vi "Velociprobe_Nanopositioner_Control_RT_2.vi"() -> ()   [LabVIEW 2015] (continued)
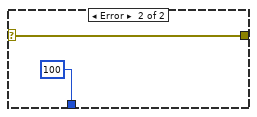
[diagram p2: hidden frame]
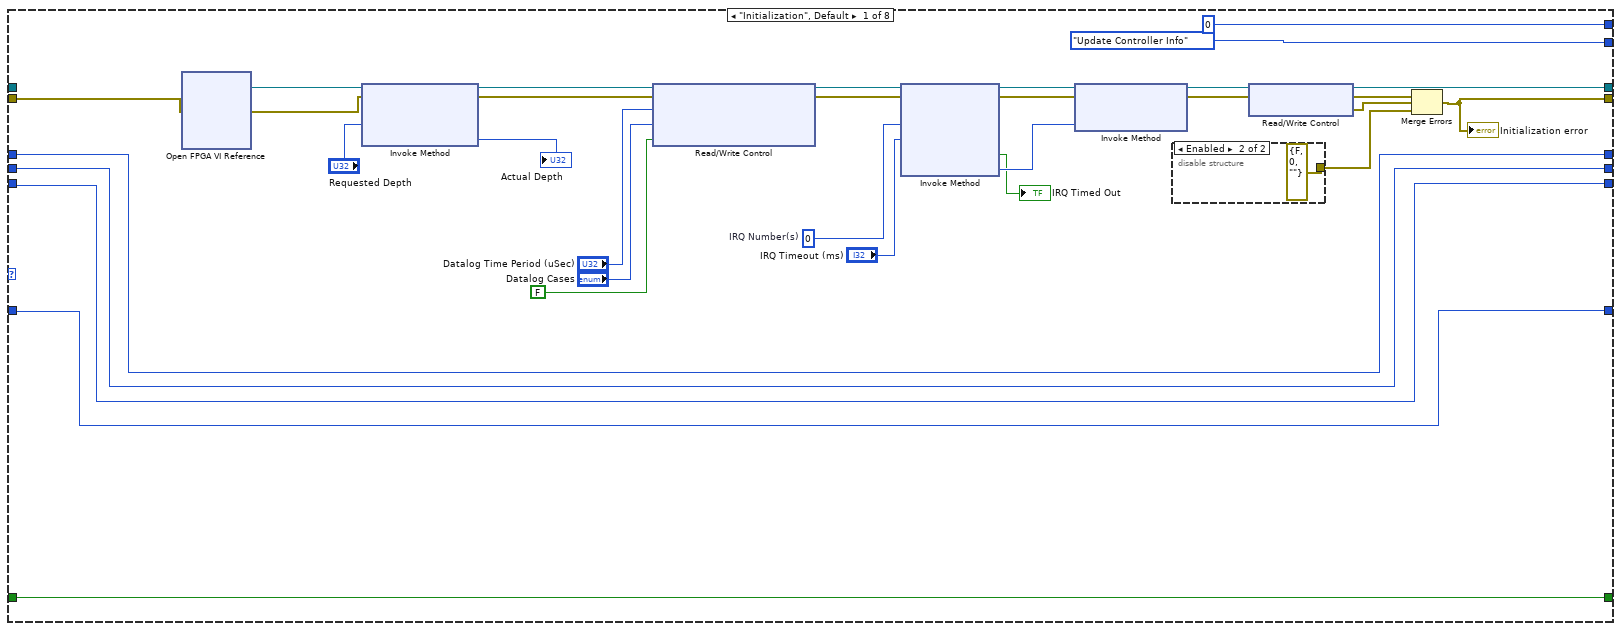
[diagram p3: hidden frame]
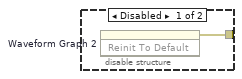
[diagram p4: hidden frame]
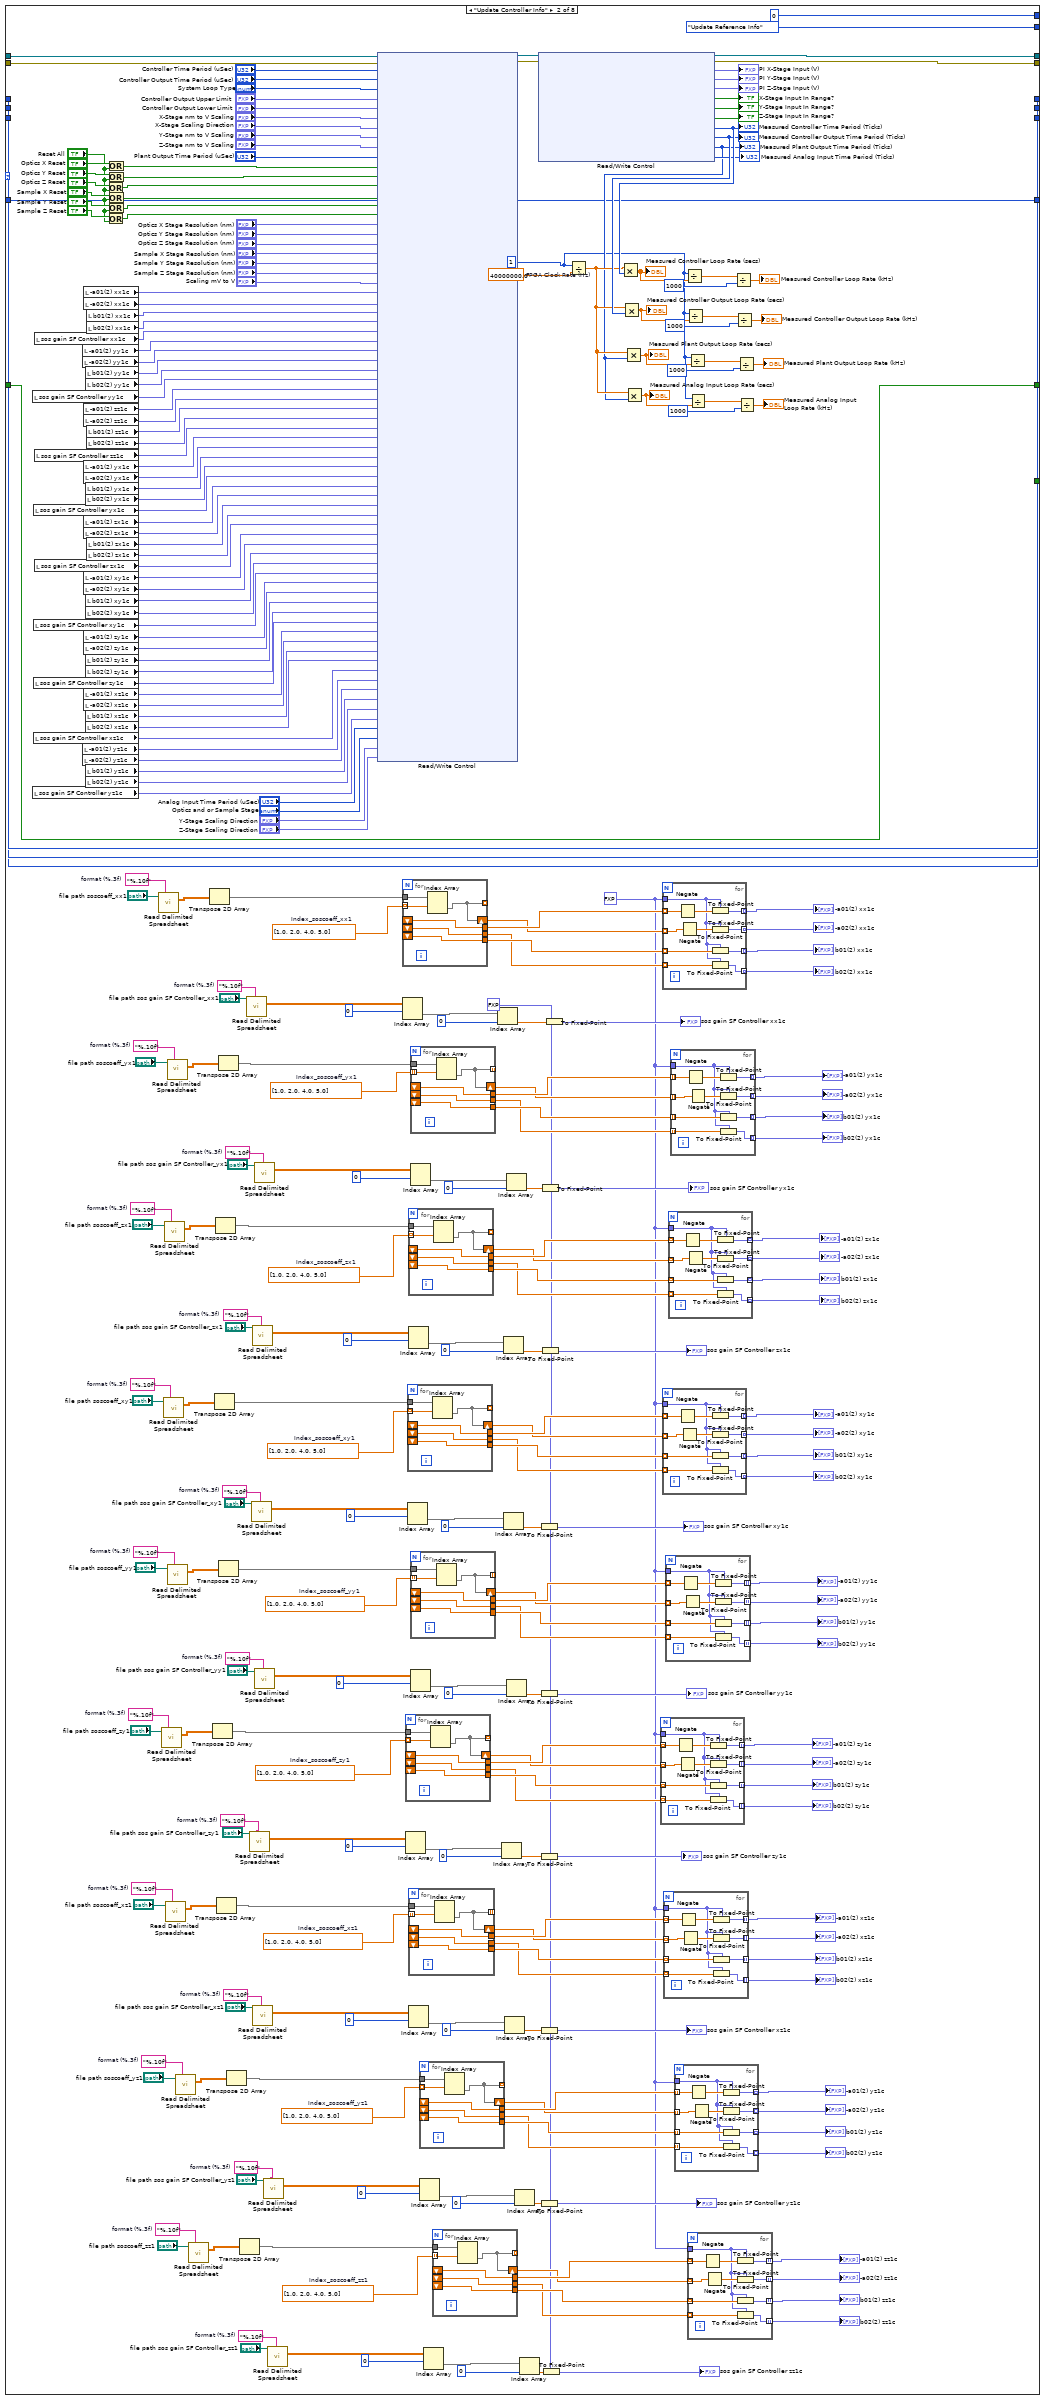
[diagram p5: hidden frame]
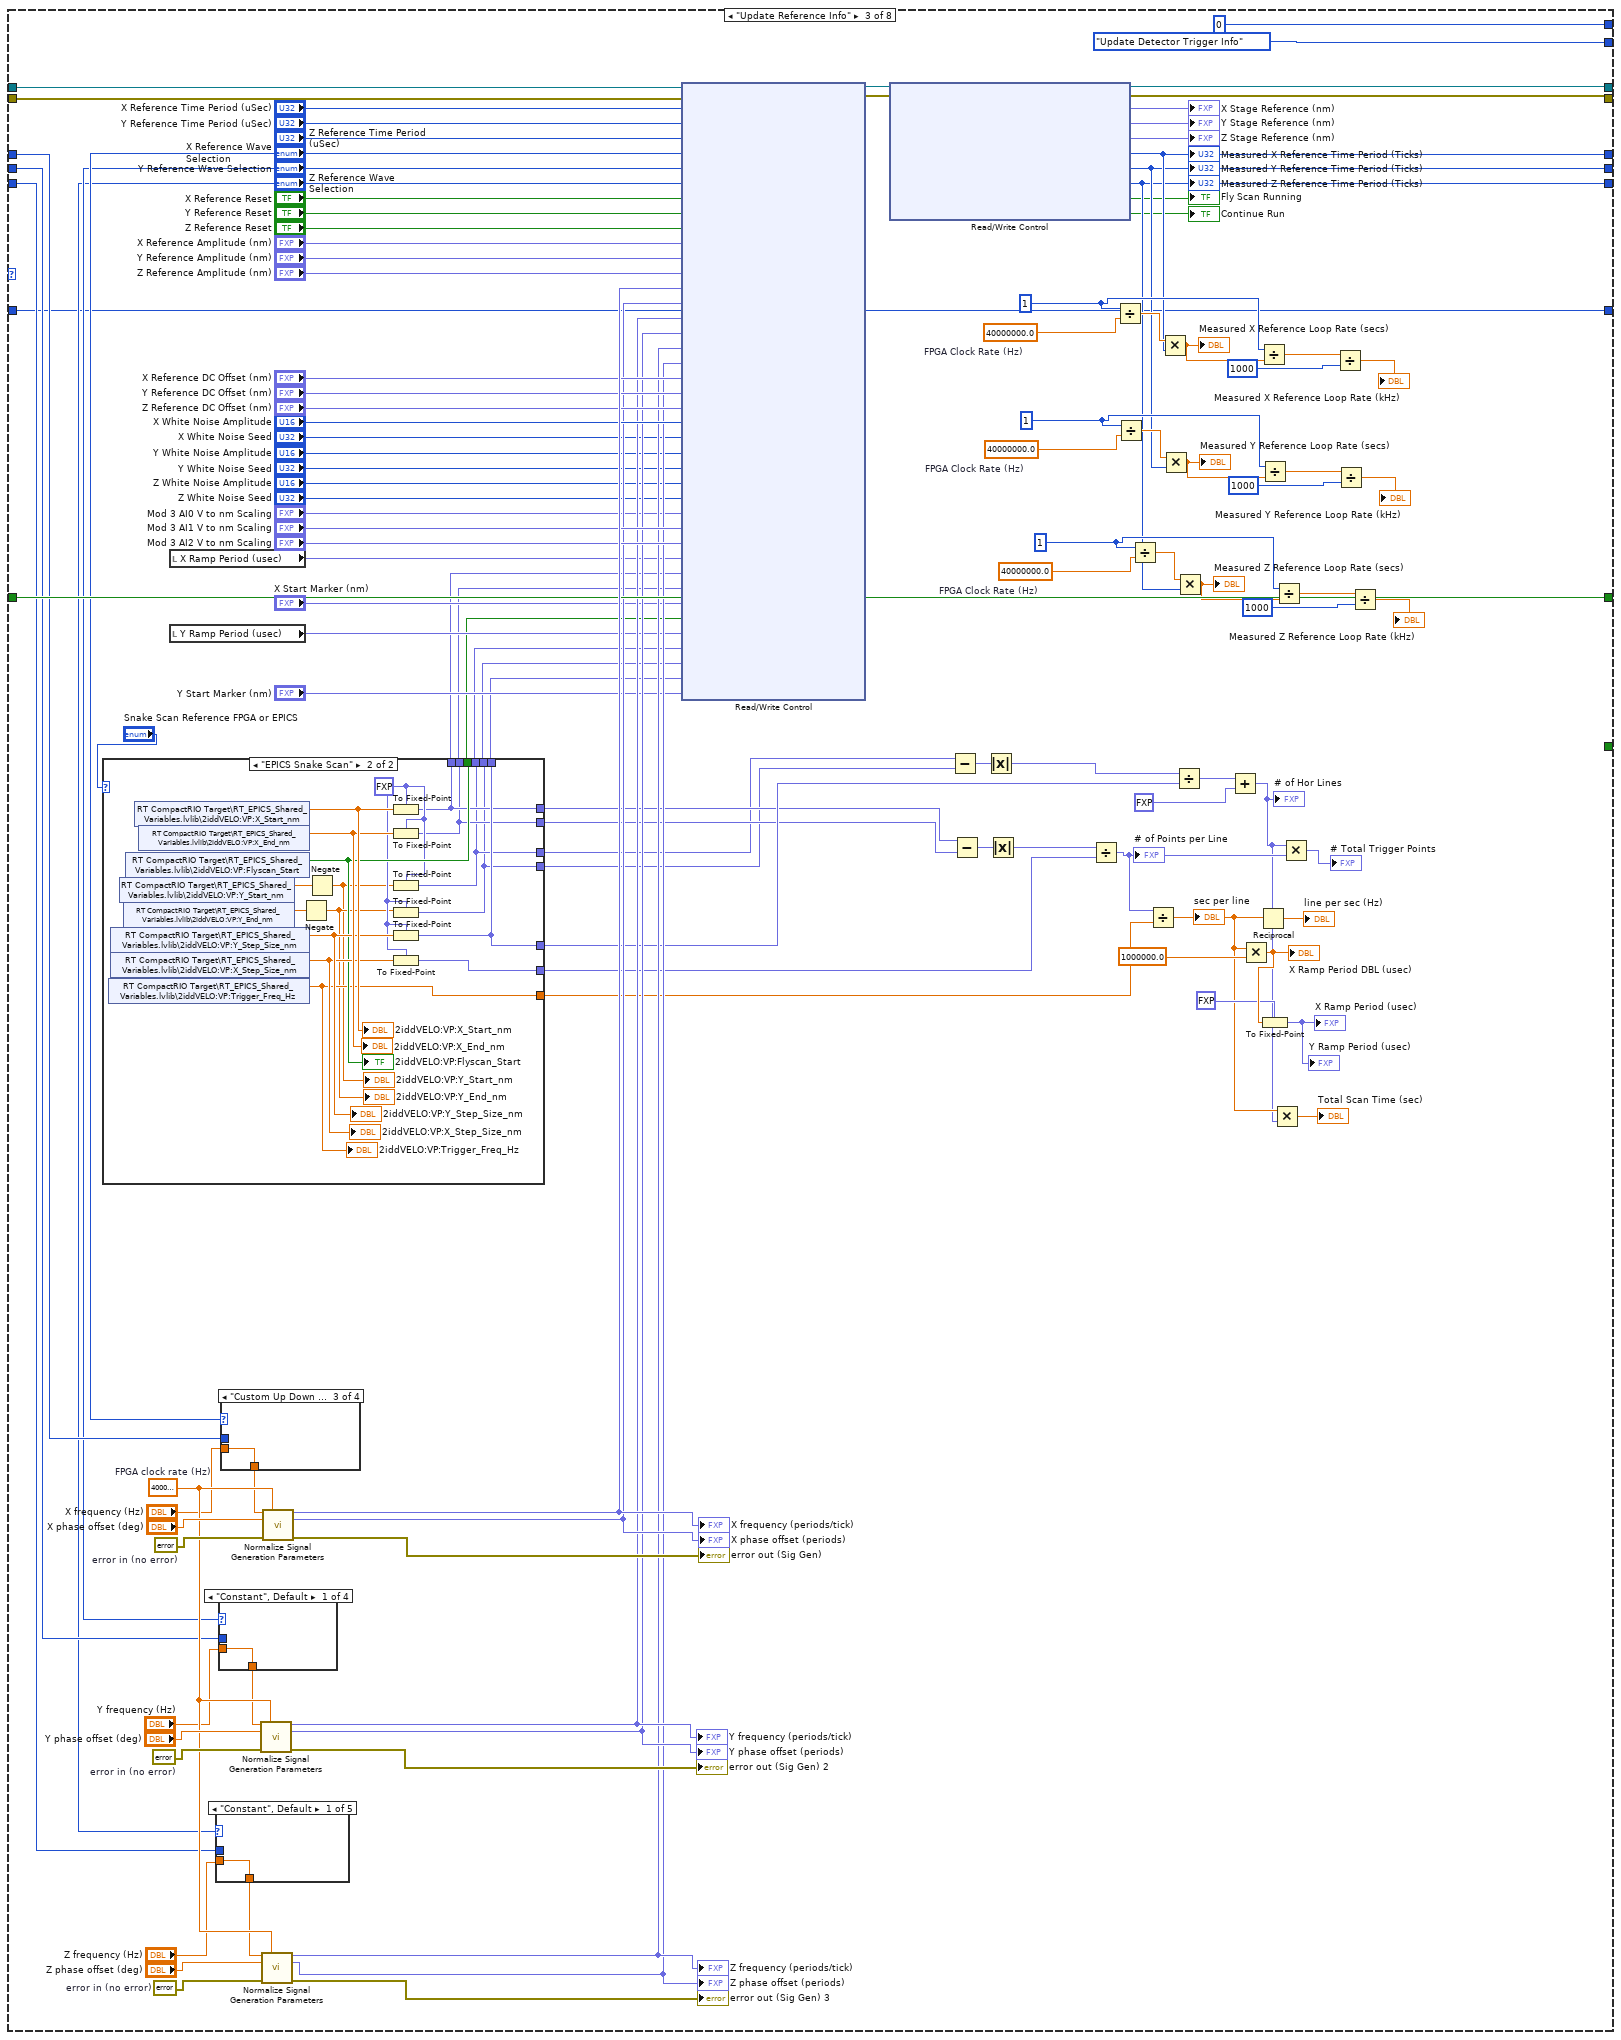
[diagram p6: hidden frame]
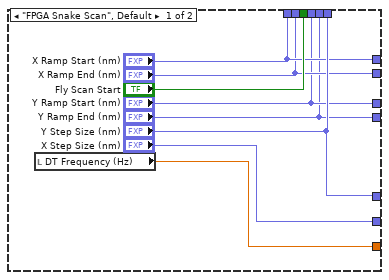
[diagram p7: hidden frame]
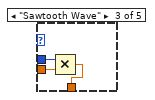
[diagram p9: hidden frame]
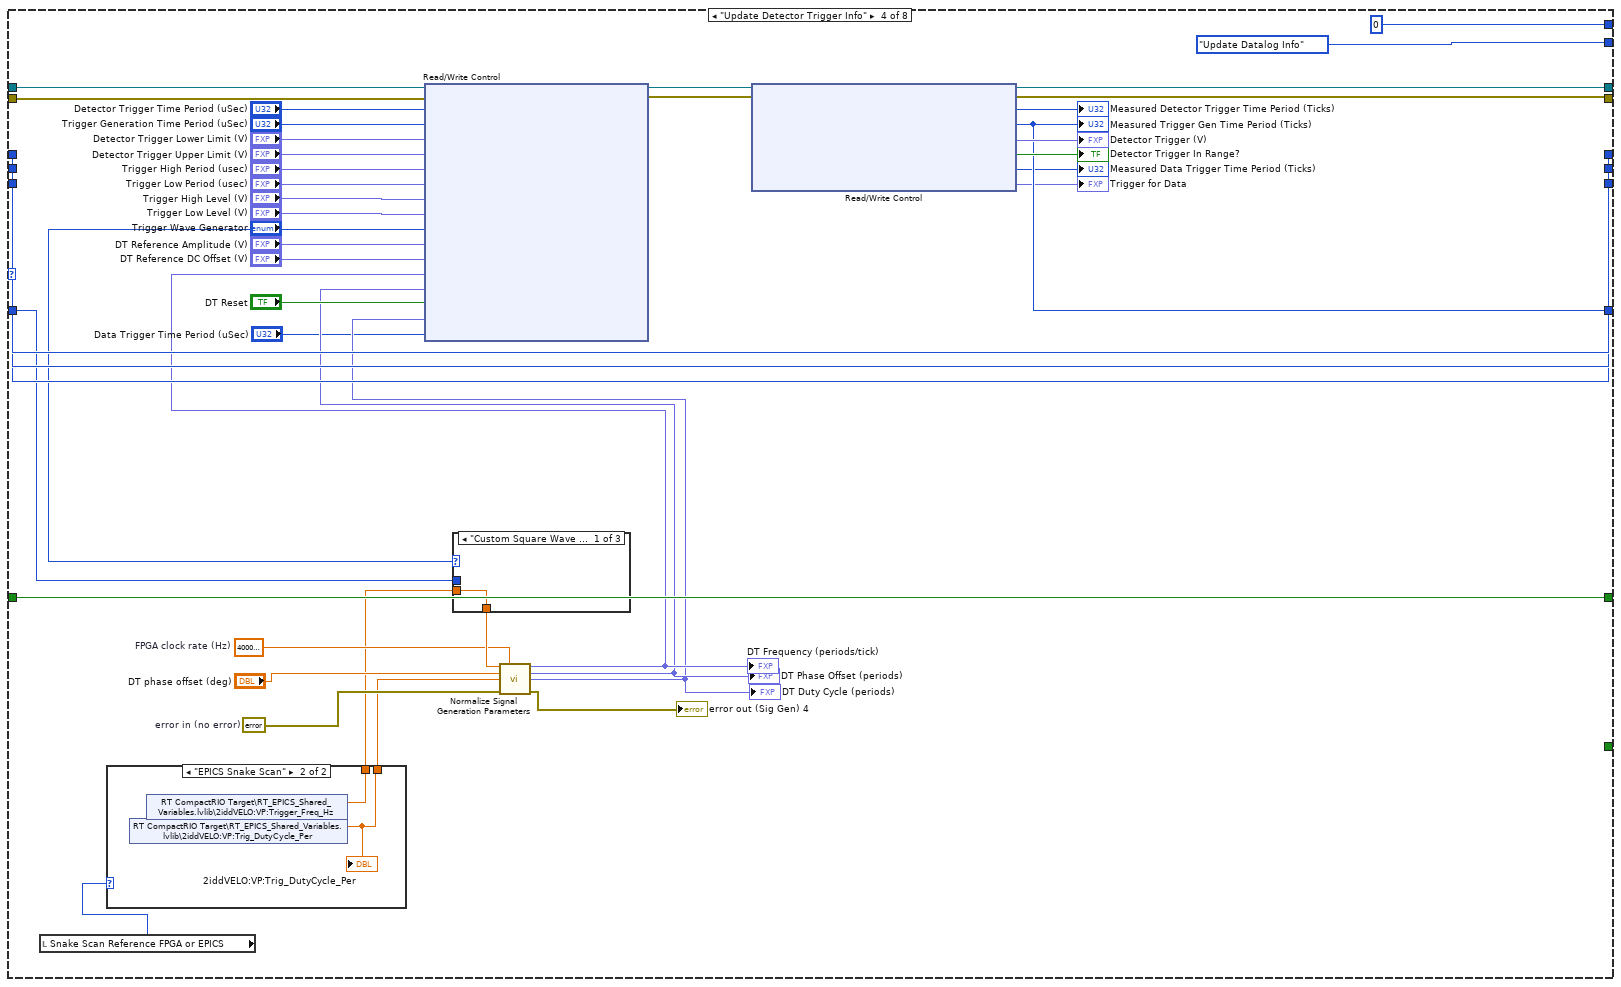
[diagram p18: hidden frame]
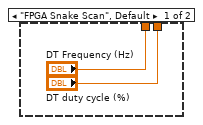
[diagram p19: hidden frame]
        n246 = xnode "Read/Write Control"("FPGA VI Reference In"=w539, "error in"=w538) -> ("FPGA VI Reference Out"=w536:refnum<k20>, "error out"=w537:errorcluster, "X Stage Reference (nm)"=→"X Stage Reference (nm)":fxp<+/-,58,25>, "Y Stage Reference (nm)"=→"Y Stage Reference (nm)":fxp<+/-,58,25>, "Z Stage Reference (nm)"=→"Z Stage Reference (nm)":fxp<+/-,58,25>, "Measured X Reference Time Period (Ticks)"=w585:u32, "Measured Y Reference Time Period (Ticks)"=w581:u32, "Measured Z Reference Time Period (Ticks)"=w580:u32, "Fly Scan Running"=→"Fly Scan Running":bool, "Continue Run"=→"Continue Run":bool)
        "Measured X Reference Time Period (Ticks)" <- w585
        "Measured Y Reference Time Period (Ticks)" <- w581
        "Measured Z Reference Time Period (Ticks)" <- w580
        n247 = Subtract(x=w532, y=w531) -> (x-y=w568:fxp<+/-,17,17>)
        n248 = Subtract(x=w534, y=w533) -> (x-y=w566:fxp<+/-,17,17>)
        n249 = Absolute Value(x=w568) -> (abs(x)=w559:fxp<+,16,16>)
        n250 = Absolute Value(x=w566) -> (abs(x)=w565:fxp<+,16,16>)
        n251 = Divide(x=w565, y=w543) -> (x/y=w563:fxp<+/-,33,17>)
        "# of Points per Line" <- w563
        n252 = Divide(x=w631, y=w637) -> (x/y=w632:dbl)
        n253 = Divide(x=w609, y=w615) -> (x/y=w610:dbl)
        n254 = Divide(x=w602, y=w608) -> (x/y=w603:dbl)
        n255 = Divide(x=w563, y=w542) -> (x/y=w555:dbl)
        "sec per line" <- w555
        n256 = Multiply(x=w632, y=w585) -> (x*y=w636:dbl)
        "Measured X Reference Loop Rate (secs)" <- w636
        n257 = Multiply(x=w610, y=w581) -> (x*y=w614:dbl)
        "Measured Y Reference Loop Rate (secs)" <- w614
        n258 = Divide(x=w559, y=w535) -> (x/y=w560:fxp<+/-,33,17>)
        n259 = Multiply(x=w603, y=w580) -> (x*y=w607:dbl)
        "Measured Z Reference Loop Rate (secs)" <- w607
        n260 = Add(x=w560, y=fxp<+,16,16> 1.0) -> (x+y=w554:fxp<+/-,34,18>)
        "# of Hor Lines" <- w554
        n261 = Multiply(x=w555, y=1000000.0) -> (x*y=w558:dbl)
        "X Ramp Period DBL (usec)" <- w558
        n262 = Reciprocal(x=w555) -> (1/x=→"line per sec (Hz)":dbl)
        n263 = Divide(x=w631, y=w636) -> (x/y=w635:dbl)
        n264 = Divide(x=w609, y=w614) -> (x/y=w613:dbl)
        n265 = To Fixed-Point(fixed-point type=fxp<+,24,24> 0.0, number=w558) -> (fixed-point=→"X Ramp Period (usec)" →"Y Ramp Period (usec)":fxp<+,24,24>)
        n266 = Multiply(x=w555, y=w554) -> (x*y=→"Total Scan Time (sec)":dbl)
        n267 = Divide(x=w602, y=w607) -> (x/y=w606:dbl)
        n268 = Multiply(x=w554, y=w563) -> (x*y=→"# Total Trigger Points":fxp<+/-,64,34>)
        n269 = Divide(x=w635, y=1000) -> (x/y=→"Measured X Reference Loop Rate (kHz)":dbl)
        n270 = Divide(x=w613, y=1000) -> (x/y=→"Measured Y Reference Loop Rate (kHz)":dbl)
        n271 = Divide(x=w606, y=1000) -> (x/y=→"Measured Z Reference Loop Rate (kHz)":dbl)
      }
      frame "Update Detector Trigger Info" {
        w711 = 40000000.0  # FPGA clock rate (Hz)
        w713 = errorcluster {"status"=FALSE, "code"=0, "source"=""}  # error in (no error)
        n272 = local read "Snake Scan Reference FPGA or EPICS"() -> (w704:enum16{"FPGA Snake Scan", "EPICS Snake Scan"})
        n273 = case shown="\"EPICS Snake Scan\"" w704 {
          tunnel: ["DT Frequency (Hz)" w739] -> w703
          tunnel: ["DT duty cycle (%)" w738] -> w702
          frame "FPGA Snake Scan", Default {
          }
          frame "EPICS Snake Scan" {
            n274 = shared-variable "RT CompactRIO Target\\RT_EPICS_Shared_Variables.lvlib\\2iddVELO:VP:Trig_DutyCycle_Per"() -> (w738:dbl)  [unwired: 1 in, 1 out]
            "2iddVELO:VP:Trig_DutyCycle_Per" <- w738
            n275 = shared-variable "RT CompactRIO Target\\RT_EPICS_Shared_Variables.lvlib\\2iddVELO:VP:Trigger_Freq_Hz"() -> (w739:dbl)  [unwired: 1 in, 1 out]
          }
        }
        n276 = case shown="\"Custom Square Wave \", Default" "Trigger Wave Generator" {
          tunnel: w703 -> [w740 w741 w742]
          tunnel: [w740 w741 w742] -> w712
          tunnel: w705 -> [_ _ _]
          frame "Custom Square Wave ", Default {
          }
          frame "Square Wave 1" {
          }
          frame "Square Wave 2" {
          }
        }
        n277 = call <vilib>:"Normalize Signal Generation Parameters.vi"("frequency (Hz)"=w712, "FPGA clock rate (Hz)"=w711, "phase offset (deg)"="DT phase offset (deg)", "duty cycle (%)"=w702, "error in (no error)"=w713) -> ("frequency (periods/tick)"=w709:fxp<+,32,0>, "phase offset (periods)"=w708:fxp<+,32,0>, "duty cycle (periods)"=w707:fxp<+,32,0>, "error out"=→"error out (Sig Gen) 4":errorcluster)  [unwired: 5 in, 2 out]
        "DT Frequency (periods/tick)" <- w709
        "DT Phase Offset (periods)" <- w708
        "DT Duty Cycle (periods)" <- w707
        n278 = xnode "Read/Write Control"("FPGA VI Reference In"=w701, "error in"=w700, "Detector Trigger Time Period (uSec)"="Detector Trigger Time Period (uSec)", "Trigger Generation Time Period (uSec)"="Trigger Generation Time Period (uSec)", "Detector Trigger Lower Limit (V)"="Detector Trigger Lower Limit (V)", "Detector Trigger Upper Limit (V)"="Detector Trigger Upper Limit (V)", "Trigger High Period (usec)"="Trigger High Period (usec)", "Trigger Low Period (usec)"="Trigger Low Period (usec)", "Trigger High Level (V)"="Trigger High Level (V)", "Trigger Low Level (V)"="Trigger Low Level (V)", "Trigger Wave Generator"="Trigger Wave Generator", "DT Reference Amplitude (V)"="DT Reference Amplitude (V)", "DT Reference DC Offset (V)"="DT Reference DC Offset (V)", "DT Frequency (periods/tick)"=w709, "DT Phase Offset (periods)"=w708, "DT Reset"="DT Reset", "DT Duty Cycle (periods)"=w707, "Data Trigger Time Period (uSec)"="Data Trigger Time Period (uSec)") -> ("FPGA VI Reference Out"=w699:refnum<k20>, "error out"=w698:errorcluster)
        n279 = xnode "Read/Write Control"("FPGA VI Reference In"=w699, "error in"=w698) -> ("FPGA VI Reference Out"=w697:refnum<k20>, "error out"=w696:errorcluster, "Measured Detector Trigger Time Period (Ticks)"=→"Measured Detector Trigger Time Period (Ticks)":u32, "Measured Trigger Gen Time Period (Ticks)"=w706:u32, "Detector Trigger (V)"=→"Detector Trigger (V)":fxp<+/-,20,5>, "Detector Trigger In Range?"=→"Detector Trigger In Range?":bool, "Measured Data Trigger Time Period (Ticks)"=→"Measured Data Trigger Time Period (Ticks)":u32, "Trigger for Data"=→"Trigger for Data":fxp<+/-,58,25>)
        "Measured Trigger Gen Time Period (Ticks)" <- w706
      }
      frame "Update Datalog Info" {
        w787 = 40000000.0  # FPGA Clock Rate (Hz)
        w776 = 1
        n280 = local read "Datalog Time Period (uSec)"() -> (w774:u32)
        n281 = local read "Datalog Cases"() -> (w773:T2)
        n282 = xnode "Read/Write Control"("FPGA VI Reference In"=w748, "error in"=w747, "Datalog Time Period (uSec)"=w774, "Datalog Cases"=w773, "Timeout FPGA FIFO1"="Timeout FPGA FIFO1") -> ("FPGA VI Reference Out"=w746:refnum<k20>, "error out"=w745:errorcluster)
        n283 = xnode "Read/Write Control"("FPGA VI Reference In"=w746, "error in"=w745) -> ("FPGA VI Reference Out"=w743:refnum<k20>, "error out"=w744:errorcluster, "Measured Datalog Time Period (Ticks)"=w786:u32, "Measured Counter Time Period (Ticks)"=w784:u32, "Mod4/DIO0"=→"Mod4/DIO0":bool, "Mod4/DIO1"=→"Mod4/DIO1":bool, "Mod4/DIO2"=→"Mod4/DIO2":bool, "Mod4/DIO3"=→"Mod4/DIO3":bool, "Mod5/DIO0"=→"Mod5/DIO0":bool, "Mod5/DIO1"=→"Mod5/DIO1":bool, "Mod5/DIO2"=→"Mod5/DIO2":bool, "Mod5/DIO3"=→"Mod5/DIO3":bool, "Mod6/DIO0"=→"Mod6/DIO0":bool, "Mod6/DIO1"=→"Mod6/DIO1":bool, "Mod6/DIO2"=→"Mod6/DIO2":bool, "Mod6/DIO3"=→"Mod6/DIO3":bool, "32 bit Count Optics X"=→"32 bit Count Optics X":i32, "32 bit Count Optics  Y"=→"32 bit Count Optics  Y":i32, "32 bit Count Optics  Z"=→"32 bit Count Optics  Z":i32, "32 bit Count Sample X"=→"32 bit Count Sample X":i32, "32 bit Count Sample  Y"=→"32 bit Count Sample  Y":i32, "32 bit Count Sample  Z"=→"32 bit Count Sample  Z":i32, "Optics X Stage Displacement (nm)"=→"Optics X Stage Displacement (nm)":fxp<+/-,58,25>, "Optics Y Stage Displacement (nm)"=→"Optics Y Stage Displacement (nm)":fxp<+/-,58,25>, "Optics Z Stage Displacement (nm)"=→"Optics Z Stage Displacement (nm)":fxp<+/-,58,25>, "Sample X Stage Displacement (nm)"=→"Sample X Stage Displacement (nm)":fxp<+/-,58,25>, "Sample Y Stage Displacement (nm)"=→"Sample Y Stage Displacement (nm)":fxp<+/-,58,25>, "Sample Z Stage Displacement (nm)"=→"Sample Z Stage Displacement (nm)":fxp<+/-,58,25>)
        "Measured Datalog Time Period (Ticks)" <- w786
        "Measured Counter Time Period (Ticks)" <- w784
        n284 = Divide(x=w776, y=w787) -> (x/y=w783:dbl)
        n285 = Multiply(x=w783, y=w786) -> (x*y=w794:dbl)
        "Measured Datalog Loop Rate (secs)" <- w794
        n286 = Multiply(x=w783, y=w784) -> (x*y=w790:dbl)
        "Measured Counter Loop Rate (secs)" <- w790
        n287 = Divide(x=w776, y=w794) -> (x/y=w793:dbl)
        n288 = Divide(x=w776, y=w790) -> (x/y=w789:dbl)
        n289 = Divide(x=w793, y=1000) -> (x/y=→"Measured Datalog Loop Rate (kHz)":dbl)
        n290 = Divide(x=w789, y=1000000) -> (x/y=→"Measured Counter Loop Rate (MHz)":dbl)
      }
      frame "Check FPGA Status" {
        n291 = xnode "Read/Write Control"("FPGA VI Reference In"=w800, "error in"=w799) -> ("FPGA VI Reference Out"=w798:refnum<k20>, "error out"=w797:errorcluster, "error out (FPGA)"=w813:errorcluster, "error out (AO FPGA)"=w812:errorcluster, "FIFO Timed Out?"=→"FIFO Timed Out?":bool, "stop case"=w807:bool, "FIFO Timed Out"=w806:bool)
        "error out (FPGA)" <- w813
        "error out (AO FPGA)" <- w812
        "stop case" <- w807
        "FIFO Timed Out" <- w806
        n292 = Merge Errors "Merge Errors"(w797, w813, w812) -> (w808:errorcluster)
        n293 = Unbundle By Name "Unbundle By Name"(w808) -> ("status"=w811:bool)
        n294 = Compound Arithmetic op=OR(w811, w807, w806) -> (w809:bool)
        n295 = Bundle By Name "Bundle By Name"(cluster=w808, "status"=w809) -> (w796:errorcluster)
      }
      frame "Reading FIFO" {
        w867 = 0.0  # t0
        n296 = local read "Snake Scan Reference FPGA or EPICS"() -> (w821:enum16{"FPGA Snake Scan", "EPICS Snake Scan"})
        n297 = local read "Datalog Time Period (uSec)"() -> (w865:u32)
        n298 = xnode "Read/Write Control"("FPGA VI Reference In"=w829, "error in"=w828) -> ("FPGA VI Reference Out"=w827:refnum<k20>, "error out"=w826:errorcluster, "Number of Data Strings"=→"Number of Data Strings":i32)
        n299 = Multiply(x=1e-06, y=w865) -> (x*y=w857:dbl)
        "Datalog Time Period (sec)" <- w857
        n300 = Divide(x=1.0, y=w857) -> (x/y=w861:dbl)
        "Datalog Rate (Hz)" <- w861
        n301 = case shown="\"FPGA Snake Scan\", Default" w821 {
          tunnel: ["Write Data" w872] -> w820
          frame "FPGA Snake Scan", Default {
          }
          frame "EPICS Snake Scan" {
            n302 = shared-variable "RT CompactRIO Target\\RT_EPICS_Shared_Variables.lvlib\\2iddVELO:VP:Write_Data"() -> (w872:bool)  [unwired: 1 in, 1 out]
            "2iddVELO:VP:Write_Data" <- w872
          }
        }
        n303 = Multiply(x="FIFO Time Period", y=w861) -> (x*y=w859:dbl)
        n304 = Multiply(x=5 ("Number of Data Strings 2"), y=w859) -> (x*y=w858:dbl)
        n305 = To Unsigned Long Integer(number=w858) -> (unsigned 32bit integer=w854:u32)
        "Number of Elements" <- w854
        n306 = xnode "Invoke Method"("FPGA VI Reference In"=w827, "error in"=w826, "Number of Elements"=w854, "Timeout (ms)"="Timeout (ms)") -> ("FPGA VI Reference Out"=w825:refnum<k20>, "error out"=w824:errorcluster, "Data"=w855:fxp<+/-,58,25>[], "Elements Remaining"=→"Elements Remaining" →"Elements Remaining Waveform Chart" →"Elements Remaining Waveform Chart 3":u32)
        "Data" <- w855
        n307 = Greater?(x=w820, y=w853) -> (0:w850:bool)
        n308 = case shown="True" w850 {
          tunnel: w828 -> [w910 w913]
          tunnel: [w910 w914] -> w849
          frame False {
          }
          frame True {
            n309 = call "Data_Write.vi"("Command List"=Data_Write_Control."Initialize", "name"="name", "error initialize"=w913) -> ("error out"=w914:errorcluster)  [unwired: 4 in, 2 out]
          }
        }
        n310 = Decimate 1D Array(w855) -> (w843:fxp<+/-,58,25>[], w834:fxp<+/-,58,25>[], w833:fxp<+/-,58,25>[], w832:fxp<+/-,58,25>[], w830:fxp<+/-,58,25>[])
        n311 = Build Array(w843, w834, w833, w832, w830) -> (w868:fxp<+/-,58,25>[][])
        n312 = To Double Precision Float(number=w868) -> (double precision float=w863:dbl[][])
        n313 = Transpose 2D Array(2D array=w863) -> (transposed array=w847:dbl[][])
        n314 = case shown="True" w820 {
          tunnel: w849 -> [w902 w908]
          tunnel: [w902 w909] -> w848
          tunnel: w847 -> [_ w903]
          frame False {
          }
          frame True {
            w906 = "%8f"  # format string
            w905 = ","  # delimiter (Tab)
            n315 = Array To Spreadsheet String(delimiter (Tab)=w905, array=w903, 3:w906) -> (spreadsheet string=w904:string)
            n316 = call "Data_Write.vi"("Command List"=Data_Write_Control."Write", "Data"=w904, "error initialize"=w908) -> ("error out"=w909:errorcluster)  [unwired: 4 in, 2 out]
          }
        }
        n317 = Bundle("t0"=w867, w857, w863) -> (→"Waveform Graph 2":cluster{"t0":dbl, dbl, dbl[][]})  [unwired: 1 in]
        n318 = call "Convert to Dynamic Data"("Array"=w843) -> ("Dynamic Data Type"=w841:dynamicdata)  [unwired: 3 in]
        n319 = call "Convert to Dynamic Data2"("Array"=w834) -> ("Dynamic Data Type"=w835:dynamicdata)  [unwired: 3 in]
        n320 = call "Convert to Dynamic Data3"("Array"=w833) -> ("Dynamic Data Type"=w837:dynamicdata)  [unwired: 3 in]
        n321 = call "Convert to Dynamic Data4"("Array"=w832) -> ("Dynamic Data Type"=w836:dynamicdata)  [unwired: 3 in]
        n322 = Less?(x=w820, y=w853) -> (x < y?=w816:bool)
        n323 = call "Convert from Dynamic Data"("Dynamic Data Type"=w841) -> ("Array"=w842:dbl[])  [unwired: 3 in]
        n324 = call "Convert from Dynamic Data2"("Dynamic Data Type"=w835) -> ("Array"=w840:dbl[])  [unwired: 3 in]
        n325 = call "Convert from Dynamic Data3"("Dynamic Data Type"=w837) -> ("Array"=w839:dbl[])  [unwired: 3 in]
        n326 = call "Convert from Dynamic Data4"("Dynamic Data Type"=w836) -> ("Array"=w838:dbl[])  [unwired: 3 in]
        n327 = case shown="True" w816 {
          tunnel: w848 -> [w873 w877]
          tunnel: [w873 w876] -> w856
          frame False {
          }
          frame True {
            # "Need to remove SFTP stuff and replace with \na write to PV that file is complete --> perhaps by \nwriting full path to PV (would instigate update that \ncould be monitored and then SFTP or FTP from \npython script"
            n328 = call "Data_Write.vi"("Command List"=Data_Write_Control."Close", "error initialize"=w877) -> ("path"=w878:path, "filename"=w874:string, "error out"=w879:errorcluster)  [unwired: 5 in]
            n329 = case shown="True" "sFTP on close" {
              tunnel: w879 -> [w881 w888]
              tunnel: w878 -> [_ w886]
              tunnel: [w881 w889] -> w876
              tunnel: w874 -> [_ w887]
              frame False {
              }
              frame True {
                n330 = disable-structure shown="Disabled" {
                  disable-tunnel: [w901 _] -> w889
                  disable-tunnel: w888 -> [w900 _]
                  disable-tunnel: w887 -> [w899 _]
                  disable-tunnel: w886 -> [w898 _]
                  disable-tunnel: "remote path" -> [w897 _]
                  disable-tunnel: "dir" -> [w896 _]
                  disable-tunnel: "Connection Info." -> [w895 _]
                  disable-tunnel: "Password" -> [w894 _]
                  frame Disabled {
                    n331 = call "sFTP_send.vi"("remote path"=w897, "local path"=w898, "filename"=w899, "dir"=w896, "Connection Info."=w895, "Password"=w894, "error in (no error)"=w900) -> ("target path"=→"target path":string, "isSftpConnected"=→"isSftpConnected":bool, "Upload return"=→"Connection return":string, "Disconnect return"=→"Upload return":string, "error out"=w901:errorcluster)  [unwired: 3 in, 1 out]
                    "FTP error" <- w901
                  }
                  frame Enabled {
                  }
                }
              }
            }
          }
        }
        n332 = Bundle("Array"=w842, "Array"=w840) -> (→"XY Graph":cluster{"Array":dbl[], "Array":dbl[]})  [unwired: 1 in]
        n333 = Bundle("Array"=w839, "Array"=w838) -> (→"XY Graph 2":cluster{"Array":dbl[], "Array":dbl[]})  [unwired: 1 in]
        n334 = Merge Errors(w824, w856) -> (w823:errorcluster)
      }
      frame "Exit" {
        w927 = TRUE ("Stop")
        n335 = xnode "Invoke Method"("FPGA VI Reference In"=w921, "error in"=w920) -> ("FPGA VI Reference Out"=w919:refnum<k20>, "error out"=w918:errorcluster)
        n336 = xnode "Read/Write Control"("FPGA VI Reference In"=w919, "error in"=w918, "stop case"=TRUE) -> ("FPGA VI Reference Out"=w917:refnum<k20>, "error out"=w916:errorcluster)
        n337 = local write "Stop"(w927) -> ()
        n338 = xnode "Close FPGA VI Reference"("FPGA VI Reference In"=w917, "error in"=w916) -> ("error out"=w915:errorcluster)
      }
    }
    n339 = shared-variable ".\\Monitor SVs.lvlib\\Error Monitor"(w14) -> ()  [unwired: 1 in, 1 out]
    n340 = call "State Control.vi"("Error Input"=w14, "Input States"=w25, "Stop"="Stop") -> ("Output State"=w24:T10)  [unwired: 8 in]
    "Next State" <- w24
    n341 = node-c288(w31) -> ()  [unwired: 1 out]
    "Current state" <- w28
  }
  n342 = while {
    stop <- FALSE stop-if-true
    n343 = shared-variable ".\\Monitor SVs.lvlib\\Error Monitor"() -> (w937:errorcluster)  [unwired: 1 in, 1 out]
    n344 = case shown="No Error" w937 {
      selector: w937 -> [w944 w946]
      tunnel: [w944 w946] -> w936
      tunnel: [u32 500 ("millisecond multiple") u32 100 ("millisecond multiple")] -> w935
      frame No Error {
      }
      frame Error {
      }
    }
    "RT error" <- w936
    n345 = flat-sequence {
      tunnel: w935 -> [w939]
      tunnel: w935 -> [w941]
      frame #0 {
        n346 = Wait Until Next ms Multiple(millisecond multiple=w939) -> ()  [unwired: 1 out]
      }
      frame #1 {
        n347 = local write "Hearbeat"(TRUE) -> ()
      }
      frame #2 {
        n348 = Wait Until Next ms Multiple(millisecond multiple=w941) -> ()  [unwired: 1 out]
      }
      frame #3 {
        "Hearbeat" <- FALSE
      }
    }
  }
  n349 = node-c288(w7) -> (→"Error (RT)":errorcluster, →"Iteration Duration RT Timed-Loop":i64)
  n350 = call <vilib>:"Simple Error Handler.vi"("error in (no error)"=w2) -> ("message"=→"message":string)  [unwired: 4 in, 4 out]
